vi "FlexMag - 24-03-2023.vi"() -> ()   [LabVIEW 2018] (continued)
                              n9401 = local read "ABORT"() -> (w14872:bool)
                              n9402 = Not(x=w14873) -> (.not. x?=w14871:bool)
                              n9403 = Compound Arithmetic op=OR(w14866, w14872, w14871) -> (w14870:bool)
                            }
                          }
                        }
                      }
                      frame True {
                      }
                    }
                  }
                }
              }
              frame #35 {
                n9404 = local read "ch2-3 transfer"() -> (w14888:bool)
                n9405 = case shown="True" w14888 {
                  frame False {
                  }
                  frame True {
                    n9406 = local read "ABORT"() -> (w14889:bool)
                    n9407 = case shown="False" w14889 {
                      frame False {
                        n9408 = local write "trns 2-3 led 16"(TRUE ("trns 1-2 led 1")) -> ()
                        n9409 = Wait (ms)(milliseconds to wait=u32 100) -> ()  [unwired: 1 out]
                      }
                      frame True {
                      }
                    }
                  }
                }
              }
              frame #36 {
                n9410 = local read "ch2-3 transfer"() -> (w14892:bool)
                n9411 = case shown="True" w14892 {
                  frame False {
                  }
                  frame True {
                    n9412 = local read "ABORT"() -> (w14893:bool)
                    n9413 = case shown="False" w14893 {
                      frame False {
                        n9414 = stacked-sequence {
                          frame #0 {
                            n9415 = while {
                              i -> [w14898]
                              stop <- w14899 stop-if-true
                              n9416 = Greater Or Equal?(x=w14898, y=600) -> (x >= y?=w14896:bool)
                              n9417 = case shown="True" w14896 {
                                frame False {
                                }
                                frame True {
                                n9418 = local write "Warning Message"("Transfer process canceled!\nCH3 Left Limit Sensor problem" ("Warning Message")) -> ()
                                n9419 = local write "trns error"(TRUE ("TRNS error")) -> ()
                                }
                              }
                              n9420 = local read "CH3_Left_Limit_DI"() -> (w14894:bool)
                              n9421 = case shown="True" w14894 {
                                tunnel: [FALSE ("CH1_Trns_BP_Left_DO") TRUE ("CH1_Trns_BP_Left_DO")] -> w14895
                                frame False {
                                n9422 = Wait Until Next ms Multiple(millisecond multiple=u32 200) -> ()  [unwired: 1 out]
                                }
                                frame True {
                                }
                              }
                              n9423 = local read "ch2-3 transfer"() -> (w14902:bool)
                              n9424 = local read "ABORT"() -> (w14901:bool)
                              n9425 = Not(x=w14902) -> (.not. x?=w14900:bool)
                              n9426 = Compound Arithmetic op=OR(w14895, w14901, w14900) -> (w14899:bool)
                            }
                          }
                          frame #1 {
                            n9427 = while {
                              i -> [w14912]
                              stop <- w14913 stop-if-true
                              n9428 = Greater Or Equal?(x=w14912, y=100) -> (x >= y?=w14910:bool)
                              n9429 = case shown="True" w14910 {
                                frame False {
                                }
                                frame True {
                                n9430 = local write "Warning Message"("Transfer process canceled!\nCassette Servo couldn't be stopped" ("Warning Message")) -> ()
                                n9431 = local write "trns error"(TRUE ("TRNS error")) -> ()
                                }
                              }
                              n9432 = local read "Casette_Servo_Start/Stop DI"() -> (w14908:bool)
                              n9433 = case shown="True" w14908 {
                                tunnel: [TRUE ("CH1_Trns_BP_Left_DO") FALSE ("CH1_Trns_BP_Left_DO")] -> w14909
                                frame False {
                                }
                                frame True {
                                n9434 = Wait Until Next ms Multiple(millisecond multiple=u32 200) -> ()  [unwired: 1 out]
                                n9435 = local write "Casette_Servo_Start/Stop DO"(FALSE ("TRNS error")) -> ()
                                }
                              }
                              n9436 = local read "ch2-3 transfer"() -> (w14916:bool)
                              n9437 = local read "ABORT"() -> (w14915:bool)
                              n9438 = Not(x=w14916) -> (.not. x?=w14914:bool)
                              n9439 = Compound Arithmetic op=OR(w14909, w14915, w14914) -> (w14913:bool)
                            }
                          }
                          frame #2 {
                            n9440 = flat-sequence {
                              frame #0 {
                                n9441 = local write "Cassette_Servo_Speed AO"(0.0 ("Cassette_Servo_Speed AO")) -> ()
                                n9442 = Wait (ms)(milliseconds to wait=u32 100) -> ()  [unwired: 1 out]
                              }
                              frame #1 {
                                n9443 = local write "Cassette_Servo_Speed Set"(TRUE ("Cassette_Servo_Speed Set")) -> ()
                              }
                            }
                          }
                        }
                      }
                      frame True {
                      }
                    }
                  }
                }
              }
              frame #37 {
                n9444 = local read "ch2-3 transfer"() -> (w14926:bool)
                n9445 = case shown="True" w14926 {
                  frame False {
                  }
                  frame True {
                    n9446 = local read "ABORT"() -> (w14927:bool)
                    n9447 = case shown="False" w14927 {
                      frame False {
                        n9448 = local write "trns 2-3 led 17"(TRUE ("trns 1-2 led 1")) -> ()
                        n9449 = Wait (ms)(milliseconds to wait=u32 100) -> ()  [unwired: 1 out]
                      }
                      frame True {
                      }
                    }
                  }
                }
              }
              frame #38 {
                n9450 = local read "ch2-3 transfer"() -> (w14930:bool)
                n9451 = case shown="True" w14930 {
                  frame False {
                  }
                  frame True {
                    n9452 = local read "ABORT"() -> (w14931:bool)
                    n9453 = case shown="False" w14931 {
                      frame False {
                        n9454 = local read "target chamber"() -> (w14932:dbl)
                        n9455 = Equal?(x=w14932, y=3.0) -> (x = y?=w14933:bool)
                        n9456 = case shown="True" w14933 {
                          frame False {
                          }
                          frame True {
                            n9457 = while {
                              i -> [w14939]
                              stop <- w14940 stop-if-true
                              n9458 = Greater Or Equal?(x=w14939, y=100) -> (x >= y?=w14937:bool)
                              n9459 = case shown="True" w14937 {
                                frame False {
                                }
                                frame True {
                                n9460 = local write "Warning Message"("Transfer process canceled!\nCH3 Cassette Fix couldn't reached  to down position" ("Warning Message")) -> ()
                                n9461 = local write "trns error"(TRUE ("TRNS error")) -> ()
                                }
                              }
                              n9462 = local read "CH3_Cst_Fix_Down_DI"() -> (w14935:bool)
                              n9463 = case shown="False" w14935 {
                                tunnel: [FALSE ("CH1_Trns_BP_Left_DO") TRUE ("CH1_Trns_BP_Left_DO")] -> w14936
                                frame False {
                                n9464 = Wait Until Next ms Multiple(millisecond multiple=u32 200) -> ()  [unwired: 1 out]
                                n9465 = local write "CH3_Cst_Fix_DO"(TRUE ("TRNS error")) -> ()
                                }
                                frame True {
                                }
                              }
                              n9466 = local read "ch2-3 transfer"() -> (w14943:bool)
                              n9467 = local read "ABORT"() -> (w14942:bool)
                              n9468 = Not(x=w14943) -> (.not. x?=w14941:bool)
                              n9469 = Compound Arithmetic op=OR(w14936, w14942, w14941) -> (w14940:bool)
                            }
                          }
                        }
                      }
                      frame True {
                      }
                    }
                  }
                }
              }
              frame #39 {
                n9470 = local read "ch2-3 transfer"() -> (w14950:bool)
                n9471 = case shown="True" w14950 {
                  frame False {
                  }
                  frame True {
                    n9472 = local read "ABORT"() -> (w14951:bool)
                    n9473 = case shown="False" w14951 {
                      frame False {
                        n9474 = local write "trns 2-3 led 18"(TRUE ("trns 1-2 led 1")) -> ()
                        n9475 = Wait (ms)(milliseconds to wait=u32 100) -> ()  [unwired: 1 out]
                      }
                      frame True {
                      }
                    }
                  }
                }
              }
              frame #40 {
                n9476 = local read "ch2-3 transfer"() -> (w14954:bool)
                n9477 = case shown="True" w14954 {
                  frame False {
                  }
                  frame True {
                    n9478 = local read "ABORT"() -> (w14955:bool)
                    n9479 = case shown="False" w14955 {
                      frame False {
                        n9480 = while {
                          i -> [w14960]
                          stop <- w14961 stop-if-true
                          n9481 = Greater Or Equal?(x=w14960, y=100) -> (x >= y?=w14958:bool)
                          n9482 = case shown="True" w14958 {
                            frame False {
                            }
                            frame True {
                              n9483 = local write "Warning Message"("Transfer process canceled!\nCH2 Trns Bp Left coulnt't be closed" ("Warning Message")) -> ()
                              n9484 = local write "trns error"(TRUE ("TRNS error")) -> ()
                            }
                          }
                          n9485 = local read "CH2_Trns_BP_Left_DI"() -> (w14956:bool)
                          n9486 = case shown="True" w14956 {
                            tunnel: [TRUE ("CH1_Trns_BP_Left_DO") FALSE ("CH1_Trns_BP_Left_DO")] -> w14957
                            frame False {
                            }
                            frame True {
                              n9487 = Wait Until Next ms Multiple(millisecond multiple=u32 200) -> ()  [unwired: 1 out]
                              n9488 = local write "CH2_Trns_BP_Left_DO"(FALSE ("TRNS error")) -> ()
                            }
                          }
                          n9489 = local read "ch2-3 transfer"() -> (w14964:bool)
                          n9490 = local read "ABORT"() -> (w14963:bool)
                          n9491 = Not(x=w14964) -> (.not. x?=w14962:bool)
                          n9492 = Compound Arithmetic op=OR(w14957, w14963, w14962) -> (w14961:bool)
                        }
                      }
                      frame True {
                      }
                    }
                  }
                }
              }
              frame #41 {
                n9493 = local read "ch2-3 transfer"() -> (w14971:bool)
                n9494 = case shown="True" w14971 {
                  frame False {
                  }
                  frame True {
                    n9495 = local read "ABORT"() -> (w14972:bool)
                    n9496 = case shown="False" w14972 {
                      frame False {
                        n9497 = local write "trns 2-3 led 19"(TRUE ("trns 1-2 led 1")) -> ()
                        n9498 = Wait (ms)(milliseconds to wait=u32 100) -> ()  [unwired: 1 out]
                      }
                      frame True {
                      }
                    }
                  }
                }
              }
              frame #42 {
                n9499 = local read "ch2-3 transfer"() -> (w14975:bool)
                n9500 = case shown="True" w14975 {
                  frame False {
                  }
                  frame True {
                    n9501 = local read "ABORT"() -> (w14976:bool)
                    n9502 = case shown="False" w14976 {
                      frame False {
                        n9503 = while {
                          i -> [w14981]
                          stop <- w14982 stop-if-true
                          n9504 = Greater Or Equal?(x=w14981, y=100) -> (x >= y?=w14979:bool)
                          n9505 = case shown="True" w14979 {
                            frame False {
                            }
                            frame True {
                              n9506 = local write "Warning Message"("Transfer process canceled!\nCH3 Trns Bp Right coulnt't be closed" ("Warning Message")) -> ()
                              n9507 = local write "trns error"(TRUE ("TRNS error")) -> ()
                            }
                          }
                          n9508 = local read "CH3_Trns_BP_Right_DI"() -> (w14977:bool)
                          n9509 = case shown="True" w14977 {
                            tunnel: [TRUE ("CH1_Trns_BP_Left_DO") FALSE ("CH1_Trns_BP_Left_DO")] -> w14978
                            frame False {
                            }
                            frame True {
                              n9510 = local write "CH3_Trns_BP_Right_DO"(FALSE ("TRNS error")) -> ()
                              n9511 = Wait Until Next ms Multiple(millisecond multiple=u32 200) -> ()  [unwired: 1 out]
                            }
                          }
                          n9512 = local read "ch2-3 transfer"() -> (w14985:bool)
                          n9513 = local read "ABORT"() -> (w14984:bool)
                          n9514 = Not(x=w14985) -> (.not. x?=w14983:bool)
                          n9515 = Compound Arithmetic op=OR(w14978, w14984, w14983) -> (w14982:bool)
                        }
                      }
                      frame True {
                      }
                    }
                  }
                }
              }
              frame #43 {
                n9516 = local read "ch2-3 transfer"() -> (w14992:bool)
                n9517 = case shown="True" w14992 {
                  frame False {
                  }
                  frame True {
                    n9518 = local read "ABORT"() -> (w14993:bool)
                    n9519 = case shown="False" w14993 {
                      frame False {
                        n9520 = local write "trns 2-3 led 20"(TRUE ("trns 1-2 led 1")) -> ()
                        n9521 = Wait (ms)(milliseconds to wait=u32 100) -> ()  [unwired: 1 out]
                      }
                      frame True {
                      }
                    }
                  }
                }
              }
              frame #44 {
                n9522 = local read "ch2-3 transfer"() -> (w14996:bool)
                n9523 = case shown="True" w14996 {
                  frame False {
                  }
                  frame True {
                    n9524 = local read "ABORT"() -> (w14997:bool)
                    n9525 = case shown="False" w14997 {
                      frame False {
                        n9526 = stacked-sequence {
                          frame #0 {
                            n9527 = local read "ch2-3 transfer"() -> (w14998:bool)
                            n9528 = case shown="True" w14998 {
                              frame False {
                              }
                              frame True {
                                n9529 = local write "CH2_Trns_GV_Open_DO"(FALSE ("trns clear")) -> ()
                              }
                            }
                          }
                          frame #1 {
                            n9530 = while {
                              i -> [w15004]
                              stop <- w15005 stop-if-true
                              n9531 = Greater Or Equal?(x=w15004, y=600) -> (x >= y?=w15002:bool)
                              n9532 = case shown="True" w15002 {
                                frame False {
                                }
                                frame True {
                                n9533 = local write "Warning Message"("Transfer process canceled!\nCH2-CH3 Trns GV couldn't be closed" ("Warning Message")) -> ()
                                n9534 = local write "trns error"(TRUE ("TRNS error")) -> ()
                                }
                              }
                              n9535 = local read "CH2_Trns_Gv_Close_DI"() -> (w15000:bool)
                              n9536 = case shown="False" w15000 {
                                tunnel: [FALSE ("CH1_Trns_BP_Left_DO") TRUE ("CH1_Trns_BP_Left_DO")] -> w15001
                                frame False {
                                n9537 = local write "CH2_Trns_GV_Close_DO"(TRUE ("TRNS error")) -> ()
                                n9538 = Wait Until Next ms Multiple(millisecond multiple=u32 200) -> ()  [unwired: 1 out]
                                }
                                frame True {
                                }
                              }
                              n9539 = local read "ch2-3 transfer"() -> (w15008:bool)
                              n9540 = local read "ABORT"() -> (w15007:bool)
                              n9541 = Not(x=w15008) -> (.not. x?=w15006:bool)
                              n9542 = Compound Arithmetic op=OR(w15001, w15007, w15006) -> (w15005:bool)
                            }
                          }
                        }
                      }
                      frame True {
                      }
                    }
                  }
                }
              }
              frame #45 {
                n9543 = local read "ch2-3 transfer"() -> (w15015:bool)
                n9544 = case shown="True" w15015 {
                  frame False {
                  }
                  frame True {
                    n9545 = local read "ABORT"() -> (w15016:bool)
                    n9546 = case shown="False" w15016 {
                      frame False {
                        n9547 = local write "trns 2-3 led 21"(TRUE ("trns 1-2 led 1")) -> ()
                        n9548 = Wait (ms)(milliseconds to wait=u32 100) -> ()  [unwired: 1 out]
                      }
                      frame True {
                      }
                    }
                  }
                }
              }
              frame #46 {
                n9549 = local read "ch2-3 transfer"() -> (w15019:bool)
                n9550 = case shown="True" w15019 {
                  frame False {
                  }
                  frame True {
                    n9551 = local read "ABORT"() -> (w15020:bool)
                    n9552 = case shown="False" w15020 {
                      frame False {
                        n9553 = local read "target chamber"() -> (w15021:dbl)
                        n9554 = Equal?(x=w15021, y=3.0) -> (x = y?=w15022:bool)
                        n9555 = case shown="True" w15022 {
                          frame False {
                          }
                          frame True {
                            n9556 = stacked-sequence {
                              frame #0 {
                                n9557 = local read "ch2-3 transfer"() -> (w15024:bool)
                                n9558 = case shown="True" w15024 {
                                frame False {
                                }
                                frame True {
                                n9559 = local write "CH3_PetCool_Up_DO"(FALSE ("trns clear")) -> ()
                                }
                                }
                              }
                              frame #1 {
                                n9560 = while {
                                i -> [w15030]
                                stop <- w15031 stop-if-true
                                n9561 = Greater Or Equal?(x=w15030, y=300) -> (x >= y?=w15028:bool)
                                n9562 = case shown="True" w15028 {
                                frame False {
                                }
                                frame True {
                                n9563 = local write "Warning Message"("Transfer process canceled!\nCH3 Petcool couldn't be down" ("Warning Message")) -> ()
                                n9564 = local write "trns error"(TRUE ("TRNS error")) -> ()
                                }
                                }
                                n9565 = local read "CH3_PetCool_Down_DI"() -> (w15026:bool)
                                n9566 = case shown="False" w15026 {
                                tunnel: [FALSE ("CH1_Trns_BP_Left_DO") TRUE ("CH1_Trns_BP_Left_DO")] -> w15027
                                frame False {
                                n9567 = local write "CH3_PetCool_Down_DO"(TRUE ("TRNS error")) -> ()
                                n9568 = Wait Until Next ms Multiple(millisecond multiple=u32 200) -> ()  [unwired: 1 out]
                                }
                                frame True {
                                }
                                }
                                n9569 = local read "ch2-3 transfer"() -> (w15034:bool)
                                n9570 = local read "ABORT"() -> (w15033:bool)
                                n9571 = Not(x=w15034) -> (.not. x?=w15032:bool)
                                n9572 = Compound Arithmetic op=OR(w15027, w15033, w15032) -> (w15031:bool)
                                }
                              }
                            }
                          }
                        }
                      }
                      frame True {
                      }
                    }
                  }
                }
              }
              frame #47 {
                n9573 = local read "ch2-3 transfer"() -> (w15041:bool)
                n9574 = case shown="True" w15041 {
                  frame False {
                  }
                  frame True {
                    n9575 = local read "ABORT"() -> (w15042:bool)
                    n9576 = case shown="False" w15042 {
                      frame False {
                        n9577 = local write "trns 2-3 led 22"(TRUE ("trns 1-2 led 1")) -> ()
                        n9578 = Wait (ms)(milliseconds to wait=u32 100) -> ()  [unwired: 1 out]
                      }
                      frame True {
                      }
                    }
                  }
                }
              }
              frame #48 {
                n9579 = local read "ch2-3 transfer"() -> (w15045:bool)
                n9580 = case shown="True" w15045 {
                  frame False {
                  }
                  frame True {
                    n9581 = local read "ABORT"() -> (w15046:bool)
                    n9582 = case shown="False" w15046 {
                      frame False {
                        n9583 = local read "target chamber"() -> (w15048:dbl)
                        n9584 = Equal?(x=w15048, y=3.0) -> (x = y?=w15047:bool)
                        n9585 = case shown="True" w15047 {
                          frame False {
                          }
                          frame True {
                            n9586 = stacked-sequence {
                              frame #0 {
                                n9587 = local read "ch2-3 transfer"() -> (w15050:bool)
                                n9588 = case shown="True" w15050 {
                                frame False {
                                }
                                frame True {
                                n9589 = local write "CH3_SRV1_Piston_Back_DO"(FALSE ("trns clear")) -> ()
                                }
                                }
                              }
                              frame #1 {
                                n9590 = while {
                                i -> [w15056]
                                stop <- w15057 stop-if-true
                                n9591 = Greater Or Equal?(x=w15056, y=200) -> (x >= y?=w15054:bool)
                                n9592 = case shown="True" w15054 {
                                frame False {
                                }
                                frame True {
                                n9593 = local write "Warning Message"("Transfer process canceled!\nCH3 Servo Piston couldn't be forward" ("Warning Message")) -> ()
                                n9594 = local write "trns error"(TRUE ("TRNS error")) -> ()
                                }
                                }
                                n9595 = local read "CH3_SRV1_Piston_For_DI"() -> (w15052:bool)
                                n9596 = case shown="False" w15052 {
                                tunnel: [FALSE ("CH1_Trns_BP_Left_DO") TRUE ("CH1_Trns_BP_Left_DO")] -> w15053
                                frame False {
                                n9597 = local write "CH3_SRV1_Piston_For_DO"(TRUE ("TRNS error")) -> ()
                                n9598 = Wait Until Next ms Multiple(millisecond multiple=u32 200) -> ()  [unwired: 1 out]
                                }
                                frame True {
                                }
                                }
                                n9599 = local read "ch2-3 transfer"() -> (w15060:bool)
                                n9600 = local read "ABORT"() -> (w15059:bool)
                                n9601 = Not(x=w15060) -> (.not. x?=w15058:bool)
                                n9602 = Compound Arithmetic op=OR(w15053, w15059, w15058) -> (w15057:bool)
                                }
                              }
                            }
                          }
                        }
                      }
                      frame True {
                      }
                    }
                  }
                }
              }
              frame #49 {
                n9603 = local read "ch2-3 transfer"() -> (w15067:bool)
                n9604 = case shown="True" w15067 {
                  frame False {
                  }
                  frame True {
                    n9605 = local read "ABORT"() -> (w15068:bool)
                    n9606 = case shown="False" w15068 {
                      frame False {
                        n9607 = local write "trns 2-3 led 23"(TRUE ("trns 1-2 led 1")) -> ()
                        n9608 = Wait (ms)(milliseconds to wait=u32 100) -> ()  [unwired: 1 out]
                      }
                      frame True {
                      }
                    }
                  }
                }
              }
              frame #50 {
                n9609 = local read "ch2-3 transfer"() -> (w15071:bool)
                n9610 = case shown="True" w15071 {
                  frame False {
                  }
                  frame True {
                    n9611 = local read "ABORT"() -> (w15072:bool)
                    n9612 = case shown="False" w15072 {
                      frame False {
                        n9613 = disable-structure shown="Enabled" {
                          frame Disabled {
                            n9614 = stacked-sequence {
                              frame #0 {
                                n9615 = while {
                                i -> [w15077]
                                stop <- w15078 stop-if-true
                                n9616 = Greater Or Equal?(x=w15077, y=100) -> (x >= y?=w15075:bool)
                                n9617 = case shown="True" w15075 {
                                frame False {
                                }
                                frame True {
                                n9618 = local write "Warning Message"("Transfer process canceled!\nRight Slow Sensor problem" ("Warning Message")) -> ()
                                n9619 = local write "trns error"(TRUE ("TRNS error")) -> ()
                                }
                                }
                                n9620 = local read "Cnt_Right_Slow DI"() -> (w15073:bool)
                                n9621 = case shown="True" w15073 {
                                tunnel: [TRUE ("CH1_Trns_BP_Left_DO") FALSE ("CH1_Trns_BP_Left_DO")] -> w15074
                                frame False {
                                }
                                frame True {
                                n9622 = Wait Until Next ms Multiple(millisecond multiple=u32 200) -> ()  [unwired: 1 out]
                                n9623 = local write "Cnt_Right_Slow DO"(FALSE ("TRNS error")) -> ()
                                }
                                }
                                n9624 = local read "ch2-3 transfer"() -> (w15081:bool)
                                n9625 = local read "ABORT"() -> (w15080:bool)
                                n9626 = Not(x=w15081) -> (.not. x?=w15079:bool)
                                n9627 = Compound Arithmetic op=OR(w15074, w15080, w15079) -> (w15078:bool)
                                }
                              }
                              frame #1 {
                                n9628 = while {
                                i -> [w15092]
                                stop <- w15093 stop-if-true
                                n9629 = Greater Or Equal?(x=w15092, y=100) -> (x >= y?=w15090:bool)
                                n9630 = case shown="True" w15090 {
                                frame False {
                                }
                                frame True {
                                n9631 = local write "Warning Message"("Transfer process canceled!\nRight Limit Sensor problem" ("Warning Message")) -> ()
                                n9632 = local write "trns error"(TRUE ("TRNS error")) -> ()
                                }
                                }
                                n9633 = local read "Cnt_Right_Limit DI"() -> (w15088:bool)
                                n9634 = case shown="True" w15088 {
                                tunnel: [TRUE ("CH1_Trns_BP_Left_DO") FALSE ("CH1_Trns_BP_Left_DO")] -> w15089
                                frame False {
                                }
                                frame True {
                                n9635 = Wait Until Next ms Multiple(millisecond multiple=u32 200) -> ()  [unwired: 1 out]
                                n9636 = local write "Cnt_Right_Limit DO"(FALSE ("TRNS error")) -> ()
                                }
                                }
                                n9637 = local read "ch2-3 transfer"() -> (w15096:bool)
                                n9638 = local read "ABORT"() -> (w15095:bool)
                                n9639 = Not(x=w15096) -> (.not. x?=w15094:bool)
                                n9640 = Compound Arithmetic op=OR(w15089, w15095, w15094) -> (w15093:bool)
                                }
                              }
                              frame #2 {
                                n9641 = while {
                                i -> [w15107]
                                stop <- w15108 stop-if-true
                                n9642 = Greater Or Equal?(x=w15107, y=100) -> (x >= y?=w15105:bool)
                                n9643 = case shown="True" w15105 {
                                frame False {
                                }
                                frame True {
                                n9644 = local write "Warning Message"("Transfer process canceled!\nLeft Slow Sensor problem" ("Warning Message")) -> ()
                                n9645 = local write "trns error"(TRUE ("TRNS error")) -> ()
                                }
                                }
                                n9646 = local read "Cnt_Left_Slow DI"() -> (w15103:bool)
                                n9647 = case shown="True" w15103 {
                                tunnel: [TRUE ("CH1_Trns_BP_Left_DO") FALSE ("CH1_Trns_BP_Left_DO")] -> w15104
                                frame False {
                                }
                                frame True {
                                n9648 = Wait Until Next ms Multiple(millisecond multiple=u32 200) -> ()  [unwired: 1 out]
                                n9649 = local write "Cnt_Left_Slow DO"(FALSE ("TRNS error")) -> ()
                                }
                                }
                                n9650 = local read "ch2-3 transfer"() -> (w15111:bool)
                                n9651 = local read "ABORT"() -> (w15110:bool)
                                n9652 = Not(x=w15111) -> (.not. x?=w15109:bool)
                                n9653 = Compound Arithmetic op=OR(w15104, w15110, w15109) -> (w15108:bool)
                                }
                              }
                              frame #3 {
                                n9654 = while {
                                i -> [w15122]
                                stop <- w15123 stop-if-true
                                n9655 = Greater Or Equal?(x=w15122, y=100) -> (x >= y?=w15120:bool)
                                n9656 = case shown="True" w15120 {
                                frame False {
                                }
                                frame True {
                                n9657 = local write "Warning Message"("Transfer process canceled!\nLeft Limit Sensor problem" ("Warning Message")) -> ()
                                n9658 = local write "trns error"(TRUE ("TRNS error")) -> ()
                                }
                                }
                                n9659 = local read "Cnt_Left_Limit DI"() -> (w15118:bool)
                                n9660 = case shown="True" w15118 {
                                tunnel: [TRUE ("CH1_Trns_BP_Left_DO") FALSE ("CH1_Trns_BP_Left_DO")] -> w15119
                                frame False {
                                }
                                frame True {
                                n9661 = Wait Until Next ms Multiple(millisecond multiple=u32 200) -> ()  [unwired: 1 out]
                                n9662 = local write "Cnt_Left_Limit DO"(FALSE ("TRNS error")) -> ()
                                }
                                }
                                n9663 = local read "ch2-3 transfer"() -> (w15126:bool)
                                n9664 = local read "ABORT"() -> (w15125:bool)
                                n9665 = Not(x=w15126) -> (.not. x?=w15124:bool)
                                n9666 = Compound Arithmetic op=OR(w15119, w15125, w15124) -> (w15123:bool)
                                }
                              }
                            }
                          }
                          frame Enabled {
                            w15134 = FALSE ("CH4_SRV1_Piston_For_DO")
                            w15135 = FALSE ("CH4_SRV1_Piston_For_DO")
                            n9667 = local write "CH1_Right_Limit_DO"(w15135) -> ()
                            n9668 = local write "CH1_Right_Slow_DO"(w15135) -> ()
                            n9669 = local write "CH2_Right_Limit_DO"(w15135) -> ()
                            n9670 = local write "CH2_Right_Slow_DO"(w15135) -> ()
                            n9671 = local write "CH2_Left_Slow_DO"(w15135) -> ()
                            n9672 = local write "CH2_Left_Limit_DO"(w15135) -> ()
                            n9673 = Wait (ms)(milliseconds to wait=u32 2000) -> ()  [unwired: 1 out]
                            n9674 = local write "CH3_Right_Limit_DO"(w15134) -> ()
                            n9675 = local write "CH3_Right_Slow_DO"(w15134) -> ()
                            n9676 = local write "CH3_Left_Slow_DO"(w15134) -> ()
                            n9677 = local write "CH3_Left_Limit_DO"(w15134) -> ()
                            n9678 = local write "CH4_Left_Limit_DO"(w15134) -> ()
                            n9679 = local write "CH4_Left_Slow_DO"(w15134) -> ()
                          }
                        }
                      }
                      frame True {
                      }
                    }
                  }
                }
              }
              frame #51 {
                n9680 = local read "ch2-3 transfer"() -> (w15136:bool)
                n9681 = case shown="True" w15136 {
                  frame False {
                  }
                  frame True {
                    n9682 = local read "ABORT"() -> (w15137:bool)
                    n9683 = case shown="False" w15137 {
                      frame False {
                        n9684 = local write "trns 2-3 led 24"(TRUE ("trns 1-2 led 17")) -> ()
                        n9685 = Wait (ms)(milliseconds to wait=u32 100) -> ()  [unwired: 1 out]
                      }
                      frame True {
                      }
                    }
                  }
                }
              }
              frame #52 {
                n9686 = local read "ch2-3 transfer"() -> (w15140:bool)
                n9687 = case shown="True" w15140 {
                  frame False {
                  }
                  frame True {
                    n9688 = local read "ABORT"() -> (w15141:bool)
                    n9689 = case shown="False" w15141 {
                      frame False {
                        n9690 = local write "Buzzer DO"(TRUE ("trns 1-2 led 17")) -> ()
                        n9691 = Wait (ms)(milliseconds to wait=u32 3000) -> ()  [unwired: 1 out]
                        n9692 = local write "System Status"("CH2 to CH3  Transfer Completed" ("System Status")) -> ()
                      }
                      frame True {
                      }
                    }
                  }
                }
              }
              frame #53 {
                n9693 = local read "ch2-3 transfer"() -> (w15145:bool)
                n9694 = case shown="True" w15145 {
                  frame False {
                  }
                  frame True {
                    n9695 = local read "ABORT"() -> (w15146:bool)
                    n9696 = case shown="False" w15146 {
                      frame False {
                        w15147 = u16 3 items=["CH1"=1, "CH2"=2, "CH3"=3, "CH4"=4] ("cassette position selection")
                        w15148 = FALSE ("trns 1-2 led 17")
                        n9697 = Wait (ms)(milliseconds to wait=u32 1000) -> ()  [unwired: 1 out]
                        n9698 = local write "cassette position selection"(w15147) -> ()
                        n9699 = local write "ch2-3 transfer"(FALSE ("trns 1-2 led 17")) -> ()
                        n9700 = local write "Buzzer DO"(FALSE ("trns 1-2 led 17")) -> ()
                        n9701 = local write "System Status"("SEMI-AUTOMATIC MODE " ("System Status")) -> ()
                        n9702 = Not(x=w15148) -> (.not. x?=w15149:bool)
                        n9703 = local write "present location"(3.0 ("present location")) -> ()
                        n9704 = local write "casette_ch1_gui"(w15148) -> ()
                        n9705 = local write "casette_ch2_gui"(w15148) -> ()
                        n9706 = local write "casette_ch3_gui"(w15149) -> ()
                        n9707 = local write "casette_ch4_gui"(w15148) -> ()
                      }
                      frame True {
                      }
                    }
                  }
                }
              }
              frame #54 {
              }
            }
          }
          frame True {
          }
        }
      }
      frame 3 {
        n9708 = local read "ABORT"() -> (w15155:bool)
        n9709 = case shown="False" w15155 {
          frame False {
            n9710 = stacked-sequence {
              frame #0 {
                n9711 = local read "ch3-4 transfer"() -> (w15156:bool)
                n9712 = case shown="True" w15156 {
                  frame False {
                  }
                  frame True {
                    n9713 = local read "present location"() -> (w15159:dbl)
                    n9714 = Wait (ms)(milliseconds to wait=u32 100) -> ()  [unwired: 1 out]
                    n9715 = Equal?(x=w15159, y=3.0) -> (x = y?=w15160:bool)
                    n9716 = case shown="True" w15160 {
                      frame False {
                        n9717 = local write "trns error"(TRUE ("TRNS error")) -> ()
                        n9718 = local write "Warning Message"("Transfer process canceled!\nCassette is not in CH3" ("Warning Message")) -> ()
                      }
                      frame True {
                        n9719 = local write "System Status"("CH3 to CH4  Transfer in Progress" ("System Status")) -> ()
                      }
                    }
                  }
                }
              }
              frame #1 {
                n9720 = local read "ch3-4 transfer"() -> (w15164:bool)
                n9721 = case shown="True" w15164 {
                  frame False {
                  }
                  frame True {
                    n9722 = stacked-sequence {
                      frame #0 {
                        n9723 = local read "ABORT"() -> (w15165:bool)
                        n9724 = case shown="False" w15165 {
                          frame False {
                            n9725 = local write "trns pre check"(TRUE ("trns pre check")) -> ()
                          }
                          frame True {
                          }
                        }
                      }
                      frame #1 {
                        n9726 = Wait (ms)(milliseconds to wait=u32 1000) -> ()  [unwired: 1 out]
                      }
                      frame #2 {
                        n9727 = while {
                          i -> [w15173]
                          stop <- w15170 stop-if-true
                          # "10 min"
                          n9728 = local read "trns pre check"() -> (w15177:bool)
                          n9729 = local read "ch3-4 transfer"() -> (w15169:bool)
                          n9730 = local read "ABORT"() -> (w15171:bool)
                          n9731 = Greater Or Equal?(x=w15173, y=u32 2000 ("millisecond multiple")) -> (x >= y?=w15172:bool)
                          n9732 = Not(x=w15177) -> (.not. x?=w15176:bool)
                          n9733 = Not(x=w15169) -> (.not. x?=w15168:bool)
                          n9734 = Compound Arithmetic op=OR(w15172, w15176, w15171, w15168) -> (w15170:bool)
                          n9735 = Wait Until Next ms Multiple(millisecond multiple=u32 300) -> ()  [unwired: 1 out]
                        }
                      }
                    }
                  }
                }
              }
              frame #2 {
                n9736 = local read "ch3-4 transfer"() -> (w15178:bool)
                n9737 = case shown="True" w15178 {
                  frame False {
                  }
                  frame True {
                    n9738 = local read "trns V?"() -> (w15179:bool)
                    n9739 = case shown="False" w15179 {
                      frame False {
                        n9740 = stacked-sequence {
                          frame #0 {
                            n9741 = local read "ABORT"() -> (w15180:bool)
                            n9742 = case shown="False" w15180 {
                              frame False {
                                w15182 = FALSE ("CH1_CH_ATM_DO")
                                n9743 = local write "CH3_CH_ATM_DO"(w15182) -> ()
                                n9744 = local write "CH4_CH_ATM_DO"(w15182) -> ()
                                n9745 = Wait (ms)(milliseconds to wait=u32 3000) -> ()  [unwired: 1 out]
                              }
                              frame True {
                              }
                            }
                          }
                          frame #1 {
                            n9746 = while {
                              i -> [w15185]
                              stop <- w15186 stop-if-true
                              n9747 = Greater Or Equal?(x=w15185, y=200) -> (x >= y?=w15183:bool)
                              n9748 = case shown="True" w15183 {
                                frame False {
                                }
                                frame True {
                                n9749 = local write "Warning Message"("Transfer process canceled!\nChambers should be on Atmosphere Pressure" ("Warning Message")) -> ()
                                n9750 = local write "trns error"(TRUE ("TRNS error")) -> ()
                                }
                              }
                              n9751 = local read "CH3_CH_ATM_DI"() -> (w15190:bool)
                              n9752 = local read "CH4_CH_ATM_DI"() -> (w15189:bool)
                              n9753 = local read "ch3-4 transfer"() -> (w15192:bool)
                              n9754 = local read "ABORT"() -> (w15193:bool)
                              n9755 = Not(x=w15192) -> (.not. x?=w15191:bool)
                              n9756 = And(x=w15190, y=w15189) -> (x .and. y?=w15188:bool)
                              n9757 = Compound Arithmetic op=OR(w15188, w15193, w15191) -> (w15186:bool)
                              n9758 = Wait Until Next ms Multiple(millisecond multiple=u32 300) -> ()  [unwired: 1 out]
                            }
                          }
                        }
                      }
                      frame True {
                        n9759 = local read "ch3 ch pg torr"() -> (w15202:dbl)
                        n9760 = local read "ch4 ch pg torr"() -> (w15199:dbl)
                        n9761 = Greater Or Equal?(x=w15202, y=0.5) -> (x >= y?=w15198:bool)
                        n9762 = Greater Or Equal?(x=w15199, y=0.5) -> (x >= y?=w15197:bool)
                        n9763 = Or(x=w15198, y=w15197) -> (x .or. y?=w15196:bool)
                        n9764 = local write "trns error"(w15196) -> ()
                      }
                    }
                  }
                }
              }
              frame #3 {
                n9765 = local read "ch3-4 transfer"() -> (w15203:bool)
                n9766 = case shown="True" w15203 {
                  frame False {
                  }
                  frame True {
                    n9767 = local read "ABORT"() -> (w15204:bool)
                    n9768 = case shown="False" w15204 {
                      frame False {
                        n9769 = while {
                          i -> [w15209]
                          stop <- w15210 stop-if-true
                          n9770 = Greater Or Equal?(x=w15209, y=100) -> (x >= y?=w15207:bool)
                          n9771 = case shown="True" w15207 {
                            frame False {
                            }
                            frame True {
                              n9772 = local write "trns error"(TRUE ("TRNS error")) -> ()
                              n9773 = local write "Warning Message"("Transfer process canceled!\nCH3 Trns BP Left couln't be opened" ("Warning Message")) -> ()
                            }
                          }
                          n9774 = local read "CH3_Trns_BP_Left_DI"() -> (w15206:bool)
                          n9775 = case shown="False" w15206 {
                            tunnel: [FALSE ("CH1_Trns_BP_Left_DO") TRUE ("CH1_Trns_BP_Left_DO")] -> w15205
                            frame False {
                              n9776 = Wait Until Next ms Multiple(millisecond multiple=u32 200) -> ()  [unwired: 1 out]
                              n9777 = local write "CH3_Trns_BP_Left_DO"(TRUE ("CH1_Trns_BP_Left_DO")) -> ()
                            }
                            frame True {
                            }
                          }
                          n9778 = local read "ch3-4 transfer"() -> (w15213:bool)
                          n9779 = local read "ABORT"() -> (w15212:bool)
                          n9780 = Not(x=w15213) -> (.not. x?=w15211:bool)
                          n9781 = Compound Arithmetic op=OR(w15205, w15212, w15211) -> (w15210:bool)
                        }
                      }
                      frame True {
                      }
                    }
                  }
                }
              }
              frame #4 {
                n9782 = local read "ch3-4 transfer"() -> (w15220:bool)
                n9783 = case shown="True" w15220 {
                  frame False {
                  }
                  frame True {
                    n9784 = local read "ABORT"() -> (w15221:bool)
                    n9785 = case shown="False" w15221 {
                      frame False {
                        n9786 = local write "trns 3-4 led 1"(TRUE ("trns 1-2 led 1")) -> ()
                        n9787 = Wait (ms)(milliseconds to wait=u32 100) -> ()  [unwired: 1 out]
                      }
                      frame True {
                      }
                    }
                  }
                }
              }
              frame #5 {
                n9788 = local read "ch3-4 transfer"() -> (w15224:bool)
                n9789 = case shown="True" w15224 {
                  frame False {
                  }
                  frame True {
                    n9790 = local read "ABORT"() -> (w15225:bool)
                    n9791 = case shown="False" w15225 {
                      frame False {
                        n9792 = while {
                          i -> [w15230]
                          stop <- w15231 stop-if-true
                          n9793 = Greater Or Equal?(x=w15230, y=100) -> (x >= y?=w15228:bool)
                          n9794 = case shown="True" w15228 {
                            frame False {
                            }
                            frame True {
                              n9795 = local write "trns error"(TRUE ("TRNS error")) -> ()
                              n9796 = local write "Warning Message"("Transfer process canceled!\nCH4 Trns BP Right couln't be opened" ("Warning Message")) -> ()
                            }
                          }
                          n9797 = local read "CH4_Trns_BP_Right_DI"() -> (w15227:bool)
                          n9798 = case shown="False" w15227 {
                            tunnel: [FALSE ("CH1_Trns_BP_Left_DO") TRUE ("CH1_Trns_BP_Left_DO")] -> w15226
                            frame False {
                              n9799 = Wait Until Next ms Multiple(millisecond multiple=u32 200) -> ()  [unwired: 1 out]
                              n9800 = local write "CH4_Trns_BP_Right_DO"(TRUE ("CH1_Trns_BP_Left_DO")) -> ()
                            }
                            frame True {
                            }
                          }
                          n9801 = local read "ch3-4 transfer"() -> (w15234:bool)
                          n9802 = local read "ABORT"() -> (w15233:bool)
                          n9803 = Not(x=w15234) -> (.not. x?=w15232:bool)
                          n9804 = Compound Arithmetic op=OR(w15226, w15233, w15232) -> (w15231:bool)
                        }
                      }
                      frame True {
                      }
                    }
                  }
                }
              }
              frame #6 {
                n9805 = local read "ch3-4 transfer"() -> (w15241:bool)
                n9806 = case shown="True" w15241 {
                  frame False {
                  }
                  frame True {
                    n9807 = local read "ABORT"() -> (w15242:bool)
                    n9808 = case shown="False" w15242 {
                      frame False {
                        n9809 = local write "trns 3-4 led 2"(TRUE ("trns 1-2 led 1")) -> ()
                        n9810 = Wait (ms)(milliseconds to wait=u32 100) -> ()  [unwired: 1 out]
                      }
                      frame True {
                      }
                    }
                  }
                }
              }
              frame #7 {
                n9811 = local read "ch3-4 transfer"() -> (w15245:bool)
                n9812 = case shown="True" w15245 {
                  frame False {
                  }
                  frame True {
                    n9813 = local read "ABORT"() -> (w15246:bool)
                    n9814 = case shown="False" w15246 {
                      frame False {
                        n9815 = stacked-sequence {
                          frame #0 {
                            n9816 = local write "CH3_Trns_GV_Close_DO"(FALSE ("CH1_Trns_Gv_Close_DO")) -> ()
                            n9817 = Wait (ms)(milliseconds to wait=u32 100) -> ()  [unwired: 1 out]
                          }
                          frame #1 {
                            n9818 = while {
                              i -> [w15253]
                              stop <- w15254 stop-if-true
                              n9819 = Greater Or Equal?(x=w15253, y=600) -> (x >= y?=w15251:bool)
                              n9820 = case shown="True" w15251 {
                                frame False {
                                }
                                frame True {
                                n9821 = local write "trns error"(TRUE ("TRNS error")) -> ()
                                n9822 = local write "Warning Message"("Transfer process canceled!\nCH3-CH4 Trns GV couln't be opened" ("Warning Message")) -> ()
                                }
                              }
                              n9823 = local read "CH3_Trns_Gv_Open_DI"() -> (w15250:bool)
                              n9824 = case shown="False" w15250 {
                                tunnel: [FALSE ("CH1_Trns_BP_Left_DO") TRUE ("CH1_Trns_BP_Left_DO")] -> w15249
                                frame False {
                                n9825 = local write "CH3_Trns_GV_Open_DO"(TRUE ("CH1_Trns_BP_Left_DO")) -> ()
                                n9826 = Wait Until Next ms Multiple(millisecond multiple=u32 200) -> ()  [unwired: 1 out]
                                }
                                frame True {
                                }
                              }
                              n9827 = local read "ch3-4 transfer"() -> (w15257:bool)
                              n9828 = local read "ABORT"() -> (w15256:bool)
                              n9829 = Not(x=w15257) -> (.not. x?=w15255:bool)
                              n9830 = Compound Arithmetic op=OR(w15249, w15256, w15255) -> (w15254:bool)
                            }
                          }
                        }
                      }
                      frame True {
                      }
                    }
                  }
                }
              }
              frame #8 {
                n9831 = local read "ch3-4 transfer"() -> (w15264:bool)
                n9832 = case shown="True" w15264 {
                  frame False {
                  }
                  frame True {
                    n9833 = local read "ABORT"() -> (w15265:bool)
                    n9834 = case shown="False" w15265 {